vi "Martins HOT interface subtract and threshold.vi"() -> ()   [LabVIEW 2012]
uses:
  Sub VIs/Trap cluster.ctl
  <vilib>/vision/Image Controls.llb/IMAQ Image.ctl
  Sub VIs/Get measurement coordinates.vi
  <vilib>/Utility/inputDevices.llb/closeKeyboard.vi
  Sub VIs/Global variables.vi
  <vilib>/Utility/inputDevices.llb/keyboardAcquire.vi
  <vilib>/vision/driver/imaqhl.llb/IMAQ Grab Acquire.vi
  <vilib>/vision/driver/IMAQdx.llb/IMAQdx Grab.vi
  <vilib>/vision/driver/imaqll.llb/IMAQ Extract Buffer.vi
  <vilib>/Utility/file.llb/Write To Spreadsheet File (DBL).vi
  <vilib>/vision/driver/NI_Vision_Acquisition_Software.lvlib
  <vilib>/vision/NI_Vision_Development_Module.lvlib
panel:
  out "Measurement image":T1
  out "Monitoring image":T1
  in  "Apply Corrections":bool
  in  "View Licence":bool
  in  "ok":bool caption="Mark the center of \nthe spot using the \nzoom and the point\ntool, then click this \nbutton"
  in  "Stop program":bool
  in  "Updating trap cluster":bool
  out "Camera enabled":bool=TRUE
  out "SLM enabled":bool=TRUE
  in  "Run calibration":bool
  in  "Hologram generation":cluster{"Method":i32, "Iterations":i32}={"Method"=1, "Iterations"=50} {"Method" items=["Lenses & Gratings (3D)", " Gerchberg-Saxton (3D)", "Gerchberg-Saxton FFT (2D)"]}
  in  "Display hologram\nand computed \nimage plane":bool
  in  "ROI":T2={"Global Rectangle"=[709, 460, 1095, 702], "Contours"=[{"Contour Type"=0, "ROI Type"=1, "Points"=[709, 497]}, {"Contour Type"=0, "ROI Type"=1, "Points"=[1094, 460]}, {"Contour Type"=0, "ROI Type"=1, "Points"=[932, 701]}]}
  out "Monitor image":T1(plugin-control)
  in  "subtract\nbackground":bool
  in  "store \nbackground":bool
  in  "Update \nhologram\nsettings":bool
  in  "Coordinate mapping \n(Monitor to Measurement)":T3={"cZ"=1.0, "cY"=0.41527447, "cX"=-0.4158654, "sZ"=0.0, "sY"=-4.372315, "sX"=686.5264}
  in  "Transpose Measurement":bool
  out "Image\nsaturated":bool
  in  "Display ROIs":bool=TRUE
  out "Lost Frames":u32=1
  in  "Display ROIs":bool
  out "Using monitoring camera\nfor measurements":bool
  out "Global Report":T4={"Mean Value"=0.10129758, "Standard Variation"=1.6580093, "Minimal Value"=0.0, "Maximal Value"=146.0, "Area (calibrated)"=346800.0, "Area (pixels)"=346800, "%"=100.0, "Calibration Valid"=TRUE} {"Mean Value" format="%.2f"; "%" format="%.2f"; "Area (calibrated)" format="%.2f"; "Maximal Value" format="%.2f"; "Minimal Value" format="%.2f"; "Standard Variation" format="%.2f"}
  in  "Save image path":path=path "E:/David/SLM characterization/Measured data/120420 - Trapping" caption="start path"
  in  "save image":bool
  in  "Subtract \nthreshold":bool=TRUE
  in  "Edit trap cluster":bool
  in  "threshold":bool
  in  "Range":cluster{"Lower value":sgl, "Upper value":sgl}={"Lower value"=20.0, "Upper value"=255.0} {"Upper value" format="%.2f"; "Lower value" format="%.2f"}
  in  "Display data":bool
  in  "Measure \nintensities":bool
  in  "Purge data":bool
  in  "ROI size":dbl=50.0 min=2.0 step=2.0
  in  "Save data":bool
  in  "Record":bool
  out "Calculated image plane":dbl[][](graph)
  in  "G":bool[](array[boolean])=[FALSE, FALSE, FALSE]
  out "Current trap pos":T5={"X (IMAQ)"=[960.0, 563.0, 45.0], "Y (IMAQ)"=[282.0, 292.0, 975.0], "Z"=[0.0, 0.0, 0.0], "I"=[10.0, 10.0, 10.0], "Trap number"=[0, 1, 2], "ROI number"=[0, 1, 2], "Number of traps"=3, "Group"=[FALSE, FALSE, FALSE]}
  out "NI Vision error":errorcluster
  out "CUDA/SLM error":errorcluster
  in  "Cancel calibration":bool
  in  "Skip step if \ntimed out":bool
  in  "Display path":bool=TRUE
  out "Average step time (ms)":dbl=26.902770233568713
  in  "Step time \n(ms)":u32=20
  in  "Pause":bool
  in  "cancel path":bool
  out "Step skipped":bool
  in  "Path controls":T6={"follow path"=FALSE, "Step length"=0.1, "Arrive \nsimultaneously"=FALSE, "Synchronize traps"=FALSE, "Add current \npositions to path"=FALSE}
  in  "Create path":bool
  out "#":i32[](array[numeric])=[0, 1, 2]
  in  "Group \nTraps":bool
  in  "Move \nHandle":bool
  out "Displayed Hologram":u8[][](graph)
  in  "Coordinate mapping \n(IMAQ to SLM)":T3={"cZ"=1.0, "cY"=0.15274464, "cX"=0.15384616, "sZ"=0.0, "sY"=-91.72315, "sX"=-106.92308}
  in  "Transpose SLM":bool
  in  "I":dbl[](array[numeric])=[15.0, 15.0, 15.0]
  in  "Z":dbl[](array[numeric])=[0.0, 0.0, 0.0]
  in  "Max num of \nmeasurements":i32=-1
  # "Martin\nPersson 2011"
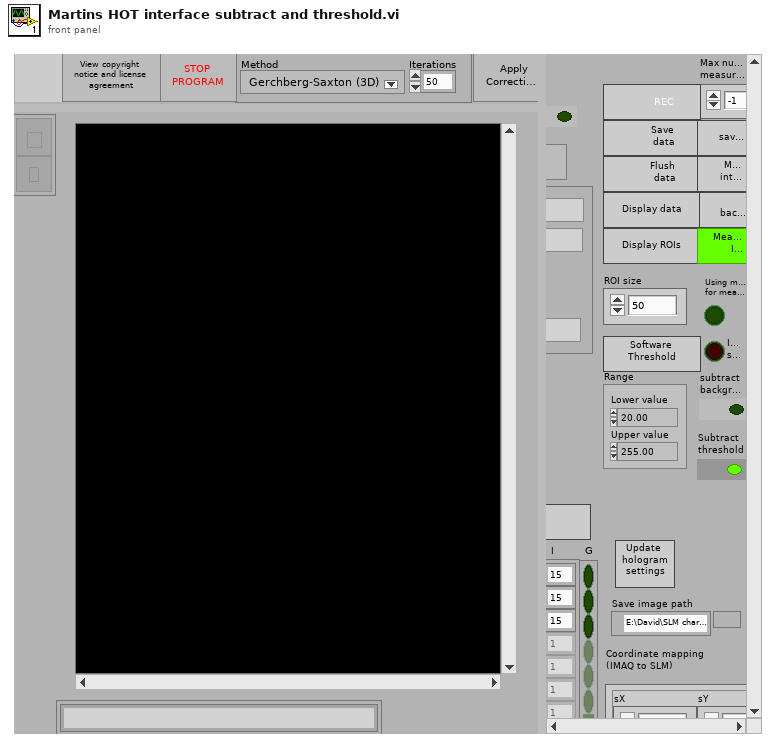
[diagram p1: front panel]
types:
  T1 = typedef "IMAQ Image.ctl" = refnum<image>
  T2 = cluster{"Global Rectangle":i32[], "Contours":cluster{"Contour Type":u32, "ROI Type":u32, "Points":i32[]}[]}
  T3 = cluster{"cZ":sgl, "cY":sgl, "cX":sgl, "sZ":sgl, "sY":sgl, "sX":sgl}
  T4 = cluster{"Mean Value":sgl, "Standard Variation":sgl, "Minimal Value":sgl, "Maximal Value":sgl, "Area (calibrated)":sgl, "Area (pixels)":u32, "%":sgl, "Calibration Valid":bool}
  T5 = typedef "Trap cluster.ctl" = cluster{"X (IMAQ)":sgl[], "Y (IMAQ)":sgl[], "Z":sgl[], "I":sgl[], "Trap number":i32[], "ROI number":i32[], "Number of traps":i32, "Group":bool[]}
  T6 = cluster{"follow path":bool, "Step length":dbl, "Arrive \nsimultaneously":bool, "Synchronize traps":bool, "Add current \npositions to path":bool}
  T7 = cluster{"CentroidX":dbl[], "CentroidY":dbl[], "I":dbl[], "Acquired Buffer Number":u32}
  T8 = enum16{"IMAQ (Camera Link)", "IMAQ ring", "IMAQdx (firewire)", "No camera"}
  T9 = typedef "IMAQdx.ctl" = refnum<k21>
  T10 = cluster{"Camera type":enum16{"IMAQ (Camera Link)", "IMAQ ring", "IMAQdx (firewire)", "No camera"}, "IMAQ Session":refnum<k11>, "IMAQdx Session":T9, "Image":T1, "Image buffers":T1[], "Camera error":errorcluster}
  T11 = typedef "Image Type" = u32
  T12 = cluster{"CentroidX":dbl[], "CentroidY":dbl[], "I":dbl[], "Acquired Buffer Number":u32}[]
  T13 = enum16{"Left Button", "Center Button", "Right Button", "Window Close"}
  T14 = typedef "ROI Descriptor" = cluster{"Global Rectangle":i32[], "Contours":cluster{"ID":enum32{"External", "Internal"}, "Type":u32, "Coordinates":i32[]}[]}
  T15 = enum16{"0", "1", "2", "3", "4", "5", "6", "7", "8", "9", "A", "B", "C", "D", "E", "F", "G", "H", "I", "J", "K", "L", "M", "N", "O", "P", "Q", "R", "S", "T", "U", "V", "W", "X", "Y", "Z", "F1", "F2", "F3", "F4", "F5", "F6", "F7", "F8", "F9", "F10", "F11", "F12", "F13", "F14", "F15", "ADD", "BACK", "BACKSLASH", "CAPITAL", "COMMA", "DECIMAL", "DELETE", "DIVIDE", "DOWN", "END", "EQUALS", "ESCAPE", "GRAVE (`)", "HOME", "INSERT", "LBRACKET", "LCONTROL", "LEFT", "L ALT", "LSHIFT", "LWIN", "MINUS", "MULTIPLY", "NEXT", "NUMLOCK", "NUMPAD_0", "NUMPAD_1", "NUMPAD_2", "NUMPAD_3", "NUMPAD_4", "NUMPAD_5", "NUMPAD_6", "NUMPAD_7", "NUMPAD_8", "NUMPAD_9", "PAUSE", "PERIOD", "PRIOR (PG UP)", "RBRACKET", "RCONTROL", "RETURN", "RIGHT", "R ALT", "RSHIFT", "RWIN", "SCROLL", "SEMICOLON", "SLASH", "SPACE", "SUBTRACT", "TAB", "UP", "ENTER (num pad)", "' (quote)"}[]
  T16 = typedef "LVRectTypeDef.ctl" = cluster{"Left":i16, "Top":i16, "Right":i16, "Bottom":i16}
  T17 = cluster{"Contour Type":u32, "ROI Type":u32, "Points":i32[]}[]
  T18 = cluster{"Contour Type":u32, "ROI Type":u32, "Points":i32[]}
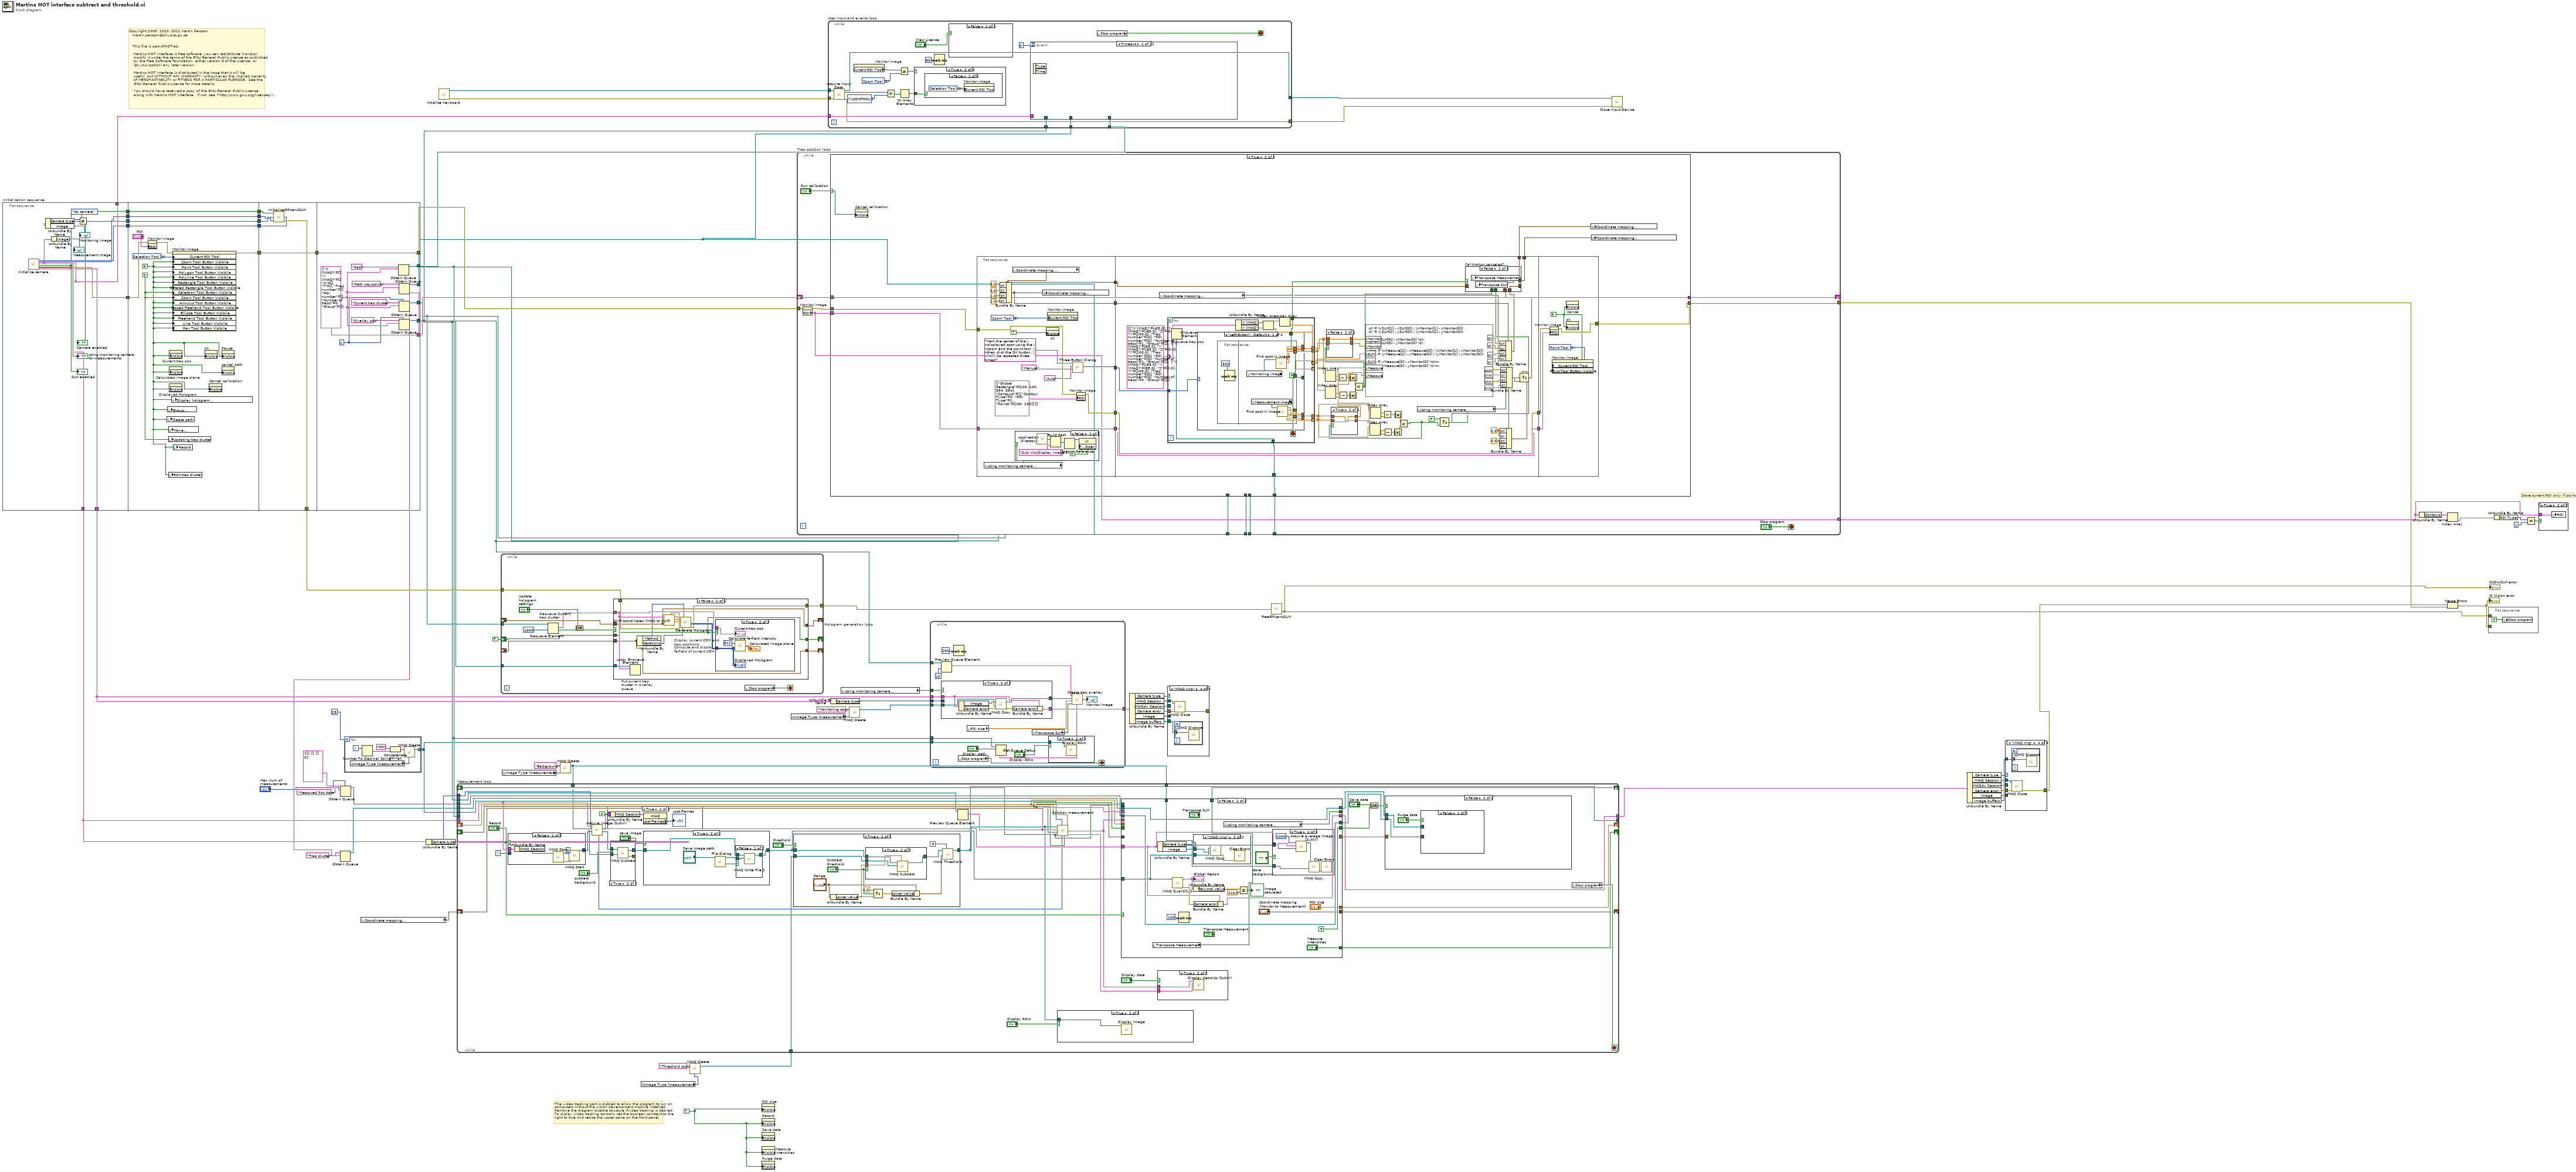
[diagram p0: block diagram]
diagram:
  w67 = TRUE ("Visible")
  # "Copyright 2009, 2010, 2011 Martin Persson \n   martin.persson@physics.gu.se\n\n\n   This file is part ofHOTlab.\n\n    Martins HOT interface is free software: you can redistribute it and/or \n    modify it under the terms of the GNU General Public License as published \n    by the Free Software Foundation, either version 3 of the License, or\n    (at your option) any later version.\n\n    Martins HOT interface is distributed in the hope that it will be \n    useful, but WITHOUT ANY WARRANTY; without even the implied warranty\n    of MERCHANTABILITY or FITNESS FOR A PARTICULAR PURPOSE.  See the\n    GNU General Public License for more details.\n\n    You should have received a copy of the GNU General Public License\n    along with Martins HOT interface.  If not, see <http://www.gnu.org/licenses/>."
  # "Store current ROI only if points"
  # "The video tracking part is disbled to allow the program to run on\ncomputers without the vision development module installed. \nRemove the diagram disable structure ifvideo tracking is desired. \nTo diplay video tracking controls, set the boolean constant to the \nright to true And resize the upper pane on the front panel."
  n1 = flat-sequence "Initialization sequence" {
    tunnel: [w82] -> w53
    tunnel: [w86] -> w52
    tunnel: [w85] -> w51
    tunnel: [w84] -> w50
    tunnel: [w83] -> w49
    tunnel: [w77] -> w26
    tunnel: [w75] -> w25
    tunnel: [w75] -> w37
    tunnel: w53 -> [w94]
    tunnel: w52 -> [w92]
    tunnel: w51 -> [w97]
    tunnel: w50 -> [w96]
    tunnel: w49 -> [w95]
    tunnel: [w94] -> w45
    tunnel: [w89] -> w44
    tunnel: [w97] -> w42
    tunnel: [w96] -> w41
    tunnel: [w95] -> w40
    tunnel: w45 -> [w100]
    tunnel: w44 -> [w103]
    tunnel: [w103] -> w43
    tunnel: w42 -> [w101]
    tunnel: w41 -> [w102]
    tunnel: w40 -> [w99]
    tunnel: [w98] -> w39
    tunnel: [w114] -> w48
    tunnel: w43 -> [w114]
    tunnel: [w112] -> w11
    tunnel: [w110] -> w47
    tunnel: [w108] -> w38
    tunnel: [w107] -> w12
    tunnel: [w104] -> w46
    frame #0 {
      n2 = call "Initialize camera.vi"() -> ("Use monitoring camera\nfor measurements"=→"Using monitoring camera\nfor measurements":bool, "Vision error out"=w86:errorcluster, "CUDA device ID"=w84:i32, "TrueFrame out"=w85:i32, "Measurement camera cluster"=w75:T10, "LUT path out"=w83:path, "SLM enabled"=w82:bool, "Monitoring camera cluster"=w77:T10)  [unwired: 3 in]
      "SLM enabled" <- w82
      n3 = Unbundle By Name(w77) -> ("Camera type"=w79:T8, "Image"=→"Monitoring image":T1)
      n4 = Unbundle By Name(w75) -> ("Image"=→"Measurement image":T1)
      n5 = Not Equal?(x=w79, y=T8."No camera") -> (x != y?=→"Camera enabled":bool)
    }
    frame #1 {
      w88 = TRUE ("ROI Tool Buttons Visibile:Zoom Tool Button Visible")
      w87 = FALSE ("ROI Tool Buttons Visibile:Zoom Tool Button Visible")
      w91 = u32 0 items=["Zoom Tool"=8, "Selection Tool"=0, "Pan Tool"=9, "Point Tool"=1, "Line Tool"=2, "Rectangle Tool"=3, "Rotated Rectangle Tool"=12, "Polyline Tool"=10, "Polygon Tool"=5, "Freehand Tool"=11, "Closed Freehand Tool"=6, "Ellipse Tool"=4, "Annulus Tool"=7] ("Current ROI Tool")
      n6 = property on="Monitor image" class="ImageControl"(error in=w92, "ROI"="ROI") -> (error out=w90:errorcluster)  [unwired: 1 in, 1 out]
      n7 = local write "Create path"(w87) -> ()
      n8 = local write "Group \nTraps"(w87) -> ()
      n9 = local write "Move \nHandle"(w87) -> ()
      n10 = local write "Updating trap cluster"(w88) -> ()
      n11 = local write "Edit trap cluster"(w87) -> ()
      n12 = property on="Current trap pos" class="Clust (strict)"("Visible"=w87) -> ()  [unwired: 2 in, 2 out]
      n13 = property on="Calculated image plane" class="IntGraph (strict)"("Visible"=w87) -> ()  [unwired: 2 in, 2 out]
      n14 = property on="Displayed Hologram" class="IntGraph (strict)"("Visible"=w87) -> ()  [unwired: 2 in, 2 out]
      n15 = local write "Display hologram\nand computed \nimage plane"(w87) -> ()
      n16 = property on="Monitor image" class="ImageControl"(error in=w90, "Current ROI Tool"=w91, "Zoom Tool Button Visibile"=w87, "Point Tool Button Visibile"=w87, "Polygon Tool Button Visibile"=w87, "Polyline Tool Button Visibile"=w87, "Rectangle Tool Button Visibile"=w87, "Rotated Rectangle Tool Button Visibile"=w87, "Selection Tool Button Visibile"=w88, "Zoom Tool Button Visibile"=w88, "Annulus Tool Button Visibile"=w87, "Closed Freehand Tool Button Visibile"=w87, "Ellipse Tool Button Visibile"=w87, "Freehand Tool Button Visibile"=w87, "Line Tool Button Visibile"=w87, "Pan Tool Button Visibile"=w87) -> (error out=w89:errorcluster)  [unwired: 1 in, 1 out]
      n17 = local write "Record"(w87) -> ()
      n18 = property on="ok" class="Bool"("Visible"=w87) -> ()  [unwired: 2 in, 2 out]
      n19 = property on="Cancel calibration" class="Bool"("Visible"=w87) -> ()  [unwired: 2 in, 2 out]
      n20 = property on="Pause" class="Bool (strict)"("Visible"=w87) -> ()  [unwired: 2 in, 2 out]
      n21 = property on="cancel path" class="Bool"("Visible"=w87) -> ()  [unwired: 2 in, 2 out]
    }
    frame #2 {
      n22 = call "InitializeGPUandSLM.vi"("TrueFrame"=w101, "deviceId"=w102, "Path to LUT file"=w99, "SLM enabled"=w100) -> ("CUDA/SLM error"=w98:errorcluster)  [unwired: 1 out]
    }
    frame #3 {
      w105 = 1 ("max queue size (-1, unlimited)")
      w104 = T5 {"X (IMAQ)"=[], "Y (IMAQ)"=[], "Z"=[], "I"=[], "Trap number"=[], "ROI number"=[], "Number of traps"=0, "Group"=[]} ("output cluster 2")
      n23 = Obtain Queue(name (unnamed)="Path", element data type=w104) -> (queue out=w112:refnum<queue>)  [unwired: 3 in, 2 out]
      n24 = Obtain Queue(name (unnamed)="Path waypoints", element data type=w104) -> (queue out=w110:refnum<queue>)  [unwired: 3 in, 2 out]
      n25 = Obtain Queue(max queue size (-1, unlimited)=w105, name (unnamed)="Current trap cluster", element data type=w104) -> (queue out=w108:refnum<queue>)  [unwired: 2 in, 2 out]
      n26 = Obtain Queue(max queue size (-1, unlimited)=w105, name (unnamed)="Overlay pos", element data type=w104) -> (queue out=w107:refnum<queue>)  [unwired: 2 in, 2 out]
    }
  }
  n27 = Obtain Queue(name (unnamed)="Trap cluster", element data type=w46) -> (queue out=w69:refnum<queue>)  [unwired: 3 in, 2 out]
  n28 = Obtain Queue(max queue size (-1, unlimited)="Max num of \nmeasurements", name (unnamed)="Measured Pos data", element data type=T7 {"CentroidX"=[], "CentroidY"=[], "I"=[], "Acquired Buffer Number"=0} ("Position data out")) -> (queue out=w71:refnum<queue>)  [unwired: 2 in, 2 out]
  n29 = for {
    N: 25 -> [_]
    tunnel: [w120] -> w10 mode=indexing
    i -> [w117]
    n30 = global read "Global variables.vi" "Image Type (measurement)"() -> (w115:T11)
    n31 = Number To Decimal String(number=w117) -> (decimal integer string=w116:string)  [unwired: 1 in]
    n32 = Concatenate Strings("ROI" ("Image Name"), w116) -> (w118:string)
    n33 = call "IMAQ Create"("Image Name"=w118, "Image Type"=w115) -> ("New Image"=w120:T1)  [unwired: 3 in, 1 out]
  }
  n34 = local read "Coordinate mapping \n(Monitor to Measurement)"() -> (w5:T3)
  n35 = Unbundle By Name(w25) -> ("Camera type"=w24:T8)
  n36 = call <vilib>:"Intialize Keyboard.vi"() -> ("error out"=w55:errorcluster, "device ID"=w73:refnum<k1>)  [unwired: 1 in, 9 out]
  n37 = while "Hologram generation loop" {
    tunnel: w38 -> [w134]
    tunnel: w12 -> [w132]
    tunnel: w39 -> [w130]
    tunnel: [w129] -> w35
    shift-right: [w128] -> _
    shift-left: _ -> [w127]
    shift-right: [w126] -> _
    shift-left: _ -> [w125]
    shift-right: [w122] -> _
    shift-left: FALSE ("Display hologram\nand computed \nimage plane") -> [w121]
    stop <- w135 stop-if-true
    n38 = Dequeue Element "Dequeue Current \ntrap cluster"(queue=w134, timeout in ms (-1)=1000) -> (element=w133:T5, timed out?=w131:bool)  [unwired: 1 in, 2 out]
    n39 = Or(x="Update \nhologram\nsettings", y=w131) -> (x .or. y?=w124:bool)
    n40 = case shown="False" w124 {
      tunnel: w127 -> [w141 _]
      tunnel: w133 -> [w145 _]
      tunnel: w132 -> [w144 _]
      tunnel: w130 -> [w143 w158]
      tunnel: [w142 w158] -> w129
      tunnel: [w141 "Coordinate mapping \n(IMAQ to SLM)"] -> w128
      tunnel: [w138 "Hologram generation"] -> w126
      tunnel: w125 -> [w138 _]
      tunnel: [w137 "Display hologram\nand computed \nimage plane"] -> w122
      tunnel: w121 -> [w137 _]
      frame False {
        n41 = Lossy Enqueue Element "Put current trap \ncluster in overlay \nqueue"(queue=w144, element=w145) -> ()  [unwired: 1 in, 4 out]
        n42 = Unbundle By Name(w138) -> ("Method"=w140:i32, "Iterations"=w139:i32)
        n43 = call "Shift coordinates (IMAQ to SLM).vi"("Trap cluster"=w145, "Coordinate mapping \n(IMAQ to SLM)"=w141) -> ("X (SLM)"=w146:sgl[], "Y (SLM)"=w149:sgl[], "Intensities"=w147:sgl[], "Z (SLM)"=w148:sgl[])  [unwired: 1 in, 1 out]
        n44 = call "Generate Hologram.vi"("x"=w146, "y"=w149, "z"=w148, "spot_intensities"=w147, "CUDA/SLM error in"=w143, "N_iterations"=w139, "method"=w140) -> ("CGH out"=w150:u8[][], "CUDA/SLM error out"=w142:errorcluster)  [unwired: 17 in, 2 out]
        n45 = case "Display current CGH and trap positions.\nCompute and display farfield of current CGH" shown="True" w137 {
          tunnel: w150 -> [_ w153]
          tunnel: w145 -> [_ w152]
          frame False {
          }
          frame True {
            n46 = call "Calculate farfield intensity.vi"("h_pSLM"=w153, "SLMsize"=512 ("Numeric")) -> ("Calculated image plane"=→"Calculated image plane":dbl[][])
            "Displayed Hologram" <- w153
            "Current trap pos" <- w152
          }
        }
      }
      frame True {
      }
    }
    n47 = local read "Stop program"() -> (w135:bool)
  }
  n48 = global read "Global variables.vi" "Image Type (measurement)"() -> (w3:T11)
  n49 = call "IMAQ Create"("Image Name"="Background", "Image Type"=w3) -> ("New Image"=w1:T1)  [unwired: 3 in, 1 out]
  n50 = global read "Global variables.vi" "Image Type (measurement)"() -> (w7:T11)
  n51 = call "IMAQ Create"("Image Name"="Threshold copy", "Image Type"=w7) -> ("New Image"=w9:T1)  [unwired: 3 in, 1 out]
  n52 = while "Measurement loop" {
    tunnel: w10 -> [w180]
    tunnel: w71 -> [w200]
    shift-right: [w199] -> _
    shift-left: _ -> [w178]
    tunnel: w69 -> [w198]
    shift-right: [w197] -> _
    shift-left: _ -> [w179]
    tunnel: [w181] -> _
    tunnel: w25 -> [w170]
    tunnel: w12 -> [w183]
    tunnel: w11 -> [_]
    tunnel: [w185] -> w29
    tunnel: w24 -> [w187]
    tunnel: w9 -> [w184]
    shift-right: [w174] -> _
    shift-left: w5 -> [w173]
    shift-right: [w165] -> _
    shift-left: _ -> [w164]
    tunnel: w1 -> [w163]
    tunnel: w1 -> [w160]
    i -> [w168]
    stop <- w201 stop-if-true
    n53 = case shown="False" "Record" {
      tunnel: w170 -> [w214 _]
      tunnel: [0 w215] -> w169
      tunnel: w168 -> [_ w215]
      frame False {
        n54 = Unbundle By Name(w214) -> ("IMAQ Session"=w213:refnum<k11>)
        n55 = call <vilib>:"IMAQ Stop.vi"("IMAQ Session In"=w213) -> ("error out"=w212:errorcluster, "IMAQ Session Out"=w211:refnum<k11>)  [unwired: 9 in]
        n56 = call <vilib>:"IMAQ Start.vi"("error in (no error)"=w212, "IMAQ Session In"=w211) -> ()  [unwired: 8 in, 2 out]
      }
      frame True {
      }
    }
    n57 = call "Acquire image (SubVI).vi"("Buffer number"=w169, "Camera type"=w187, "Measurement camera \ncluster in"=w170) -> ("Image Out"=w161:T1, "Measurement camera cluster out"=w186:T10, "Buffer Number Out"=w171:u32)  [unwired: 6 in]
    n58 = case shown="True" FALSE {
      tunnel: w186 -> [_ w207]
      frame False {
      }
      frame True {
        n59 = Unbundle By Name(w207) -> ("IMAQ Session"=w209:refnum<k11>)
        n60 = property class="IMAQ"(reference=w209) -> ("Lost Frames"=→"Lost Frames":u32)  [unwired: 1 in, 2 out]
      }
    }
    n61 = case shown="True" "subtract\nbackground" {
      tunnel: [w202 w206] -> w162
      tunnel: w161 -> [w202 w205]
      tunnel: w160 -> [_ w204]
      tunnel: [_ w203] -> _
      frame False {
      }
      frame True {
        n62 = call "IMAQ Subtract"("Image Src A"=w205, "Image Src B"=w204) -> ("Image Dst Out"=w206:T1, "error out"=w203:errorcluster)  [unwired: 5 in]
      }
    }
    n63 = case shown="True" "save image" {
      tunnel: w162 -> [w219 w224]
      tunnel: [w219 w223] -> w188
      frame False {
      }
      frame True {
        n64 = call "File Dialog"("start path"="Save image path") -> ("selected path"=w222:path, "cancelled"=w221:bool)  [unwired: 11 in, 2 out]
        n65 = case shown="False" w221 {
          tunnel: w224 -> [w227 w228]
          tunnel: [w226 w228] -> w223
          tunnel: w222 -> [w225 _]
          frame False {
            n66 = call-poly "IMAQ Write File 2"("File Path"=w225, "Image"=w227) -> ("Image Out (duplicate)"=w226:T1)  [unwired: 8 in, 1 out]
          }
          frame True {
          }
        }
      }
    }
    n67 = case shown="True" "threshold" {
      tunnel: w188 -> [w229 w237]
      tunnel: [w229 w235] -> w181
      tunnel: w184 -> [_ w230]
      frame False {
      }
      frame True {
        n68 = Unbundle By Name("Range") -> ("Lower value"=w231:sgl)
        n69 = case shown="True" "Subtract \nthreshold" {
          tunnel: w231 -> [_ w245]
          tunnel: w237 -> [w241 w244]
          tunnel: [w241 w243] -> w236
          tunnel: w230 -> [_ w242]
          frame False {
          }
          frame True {
            n70 = call "IMAQ Subtract"("Image Src A"=w244, "Constant"=w245, "Image Dst"=w242) -> ("Image Dst Out"=w243:T1)  [unwired: 4 in, 1 out]
          }
        }
        n71 = Select(t=sgl 0.0 ("Lower value"), s="Subtract \nthreshold", f=w231) -> (s? t:f=w234:sgl)
        n72 = Bundle By Name(cluster="Range", "Lower value"=w234) -> (w238:cluster{"Lower value":sgl, "Upper value":sgl})
        n73 = call "IMAQ Threshold"("Keep/Replace Value (Replace)"=FALSE, "Range"=w238, "Image Src"=w236) -> ("Image Dst Out"=w235:T1)  [unwired: 7 in, 1 out]
      }
    }
    n74 = Preview Queue Element(queue=w183) -> (element=w182:T5)  [unwired: 2 in, 3 out]
    n75 = call "Position measurement.vi"("Measure \nintensities"=w179, "ROI size"=w178, "Acquired Buffer Number"=w171, "Switch xy"=w164, "Coordinate mapping \n(Monitor to Measurement)"=w173, "ROIs"=w180, "Trap positions"=w182, "Image"=w181) -> ("Target coordinates"=w172:cluster{"X target":sgl[], "Y target":sgl[]}, "Position data out"=w176:T7)  [unwired: 1 in]
    n76 = case shown="True" "Display ROIs" {
      tunnel: w181 -> [_ w216]
      frame False {
      }
      frame True {
        n77 = call "Display Image.vi"("Image 2"=w216) -> ()  [unwired: 11 in]
      }
    }
    n78 = case shown="False" "Record" {
      tunnel: w200 -> [w266 w289]
      tunnel: [w266 w288] -> w196
      tunnel: [_ w287] -> w194
      tunnel: ["ROI size" w286] -> w199
      tunnel: w178 -> [_ w286]
      tunnel: w198 -> [w265 w285]
      tunnel: [w265 w284] -> w193
      tunnel: ["Measure \nintensities" w283] -> w197
      tunnel: w179 -> [_ w283]
      tunnel: [FALSE ("timed out?") w281] -> w190
      tunnel: w188 -> [w249 _]
      tunnel: w186 -> [w247 w280]
      tunnel: [w259 w280] -> w185
      tunnel: w182 -> [_ w279]
      tunnel: w176 -> [_ w278]
      tunnel: ["Coordinate mapping \n(Monitor to Measurement)" w277] -> w174
      tunnel: w173 -> [_ w277]
      tunnel: [w253 _] -> _
      tunnel: [w251 w276] -> w165
      tunnel: w164 -> [_ w276]
      tunnel: w163 -> [w248 _]
      frame False {
        n79 = local read "Transpose Measurement"() -> (w251:bool)
        n80 = Unbundle By Name(w247) -> ("Camera type"=w246:T8, "Image"=w252:T1)
        n81 = call "IMAQ Quantify 2"("Image"=w249) -> ("error out"=w260:errorcluster, "Global Report"=w258:T4)  [unwired: 8 in, 1 out]
        "Global Report" <- w258
        n82 = Wait (ms)(milliseconds to wait=u32 100) -> ()  [unwired: 1 out]
        n83 = case shown="\"IMAQ ring\"" w246 {
          tunnel: w249 -> [_ w275]
          tunnel: w252 -> [_ w274]
          frame "IMAQ (Camera Link)", Default {
          }
          frame "IMAQ ring" {
            n84 = call "IMAQ Copy"("Image Dst"=w274, "Image Src"=w275) -> ("error out"=w273:errorcluster)  [unwired: 4 in, 1 out]
            n85 = call <vilib>:"Clear Errors.vi"("error in (no error)"=w273) -> ()  [unwired: 6 in, 1 out]
          }
        }
        n86 = Unbundle By Name(w258) -> ("Maximal Value"=w257:sgl)
        n87 = Bundle By Name(cluster=w247, "Camera error"=w260) -> (w259:T10)
        n88 = local read "Using monitoring camera\nfor measurements"() -> (w253:bool)
        n89 = Greater Or Equal?(x=w257, y=sgl 210.0) -> (x >= y?=→"Image\nsaturated":bool)
        n90 = case shown="True" "store \nbackground" {
          tunnel: w248 -> [_ w271]
          tunnel: w247 -> [_ w270]
          tunnel: w246 -> [_ w269]
          frame False {
          }
          frame True {
            n91 = call "Acquire average image (SubVI).vi"("Camera type"=w269, "Measurement camera cluster in"=w270, "averaging time (ms)"=1000) -> ("Refnum out"=w267:T1)  [unwired: 8 in]
            n92 = call "IMAQ Copy"("Image Dst"=w271, "Image Src"=w267) -> ("error out"=w272:errorcluster)  [unwired: 4 in, 1 out]
            n93 = call <vilib>:"Clear Errors.vi"("error in (no error)"=w272) -> ()  [unwired: 6 in, 1 out]
          }
        }
      }
      frame True {
        n94 = Enqueue Element(queue=w285, element=w279) -> (queue out=w284:refnum<queue>)  [unwired: 2 in, 2 out]
        n95 = Enqueue Element(queue=w289, element=w278, timeout in ms (-1)=10000) -> (queue out=w288:refnum<queue>, timed out?=w281:bool, error out=w287:errorcluster)  [unwired: 1 in]
      }
    }
    n96 = case shown="True" "Display data" {
      tunnel: w176 -> [_ w218]
      tunnel: w172 -> [_ w217]
      frame False {
      }
      frame True {
        n97 = call "Display Cetroids (SubVI).vi"("Target coordinates"=w217, "Measurement data"=w218) -> ()  [unwired: 7 in, 3 out]
      }
    }
    n98 = Or(x="Save data", y=w190) -> (x .or. y?=w191:bool)
    n99 = case shown="False" w191 {
      tunnel: w196 -> [w291 w311]
      tunnel: w194 -> [_ w301]
      tunnel: w193 -> [w290 w300]
      frame False {
        n100 = case shown="False" "Purge data" {
          tunnel: w291 -> [_ w294]
          tunnel: w290 -> [_ w293]
          frame False {
          }
          frame True {
            n101 = Flush Queue(queue=w293) -> ()  [unwired: 1 in, 3 out]
            n102 = Flush Queue(queue=w294) -> ()  [unwired: 1 in, 3 out]
          }
        }
      }
      frame True {
        n103 = Flush Queue(queue=w311, error in (no error)=w301) -> (remaining elements=w307:T12)  [unwired: 2 out]
        n104 = Flush Queue(queue=w300, error in (no error)=w301) -> (remaining elements=w299:T5[])  [unwired: 2 out]
        n105 = for {
          tunnel: [w318] -> w310 mode=indexing
          tunnel: [w317] -> w309 mode=indexing
          tunnel: [w316] -> w302 mode=indexing
          tunnel: w307 -> [w315] mode=indexing
          tunnel: w299 -> [w314] mode=indexing
          tunnel: [w313] -> w298 mode=indexing
          tunnel: [w312] -> w297 mode=indexing
          workers-P: _ -> [_]
          n106 = Unbundle By Name(w315) -> ("CentroidX"=w318:dbl[], "CentroidY"=w317:dbl[], "Acquired Buffer Number"=w316:u32)
          n107 = Unbundle By Name(w314) -> ("X (IMAQ)"=w313:sgl[], "Y (IMAQ)"=w312:sgl[])
        }
        n108 = Transpose 2D Array(2D array=w310) -> (transposed array=w305:dbl[][])
        n109 = Transpose 2D Array(2D array=w309) -> (transposed array=w304:dbl[][])
        n110 = Transpose 2D Array(2D array=w298) -> (transposed array=w296:sgl[][])
        n111 = Transpose 2D Array(2D array=w297) -> (transposed array=w295:sgl[][])
        n112 = Build Array (concatenate)(w302, w305, w304, w296, w295) -> (w306:dbl[][])
        n113 = Transpose 2D Array(2D array=w306) -> (transposed array=w303:dbl[][])
        n114 = call-poly <vilib>:"Write To Spreadsheet File.vi"("format (%.3f)"="%.9f", "2D data"=w303) -> ()  [unwired: 6 in, 1 out]
      }
    }
    n115 = local read "Stop program"() -> (w201:bool)
  }
  n116 = property on="ROI size" class="DigNum (strict)"("Visible"=w67) -> ()  [unwired: 2 in, 2 out]
  n117 = property on="Record" class="Bool (strict)"("Visible"=w67) -> ()  [unwired: 2 in, 2 out]
  n118 = property on="Save data" class="Bool"("Visible"=w67) -> ()  [unwired: 2 in, 2 out]
  n119 = property on="Measure \nintensities" class="Bool (strict)"("Visible"=w67) -> ()  [unwired: 2 in, 2 out]
  n120 = property on="Purge data" class="Bool"("Visible"=w67) -> ()  [unwired: 2 in, 2 out]
  n121 = global read "Global variables.vi" "Image Type (measurement)"() -> (w6:T11)
  n122 = while "Trap position loop" {
    tunnel: w47 -> [w330]
    tunnel: w11 -> [w327]
    shift-right: [w329] -> _
    shift-left: w46 -> [w322]
    tunnel: w38 -> [w328]
    tunnel: w12 -> [w325]
    tunnel: [w324] -> w61
    tunnel: w48 -> [w321]
    tunnel: [w319] -> w59
    stop <- "Stop program" stop-if-true
    n123 = property on="Monitor image" class="ImageControl"(error in=w321) -> (error out=w320:errorcluster, "ROI"=w324:T2)  [unwired: 1 in, 1 out]
    n124 = case shown="True" "Run calibration" {
      selector: "Run calibration" -> [_ w534]
      tunnel: w330 -> [w356 _]
      tunnel: w322 -> [w355 w533]
      tunnel: [w334 w533] -> w329
      tunnel: w328 -> [w345 w542]
      tunnel: w327 -> [w343 _]
      tunnel: w325 -> [w340 _]
      tunnel: w324 -> [w339 w541]
      tunnel: w320 -> [w338 w538]
      tunnel: [w336 w535] -> w319
      frame False {
        n125 = case "Update trap cluster" shown="True" "Updating trap cluster" {
          tunnel: w355 -> [w358 w372]
          tunnel: [w358 w365] -> w346
          tunnel: w339 -> [_ w363]
          tunnel: w338 -> [w357 w362]
          tunnel: [w357 w361] -> w337
          frame False {
          }
          frame True {
            n126 = local read "Transpose SLM"() -> (w371:bool)
            n127 = call "Manage ROI.vi"("Switch X/Y"=w371, "Trap cluster in"=w372, "ROI in"=w363, "Group traps"="Group \nTraps") -> ("Replace ROI"=w359:bool, "ROI out"=w364:T2, "Previous ROI out"=w370:T2)
            n128 = case "Modify trap cluster for \ngroup or a single trap" shown="False" "Group \nTraps" {
              tunnel: [w382 w421] -> w365
              tunnel: w364 -> [w389 w422]
              tunnel: w372 -> [w388 w424]
              tunnel: w370 -> [_ w423]
              tunnel: "Z" -> [w387 w420]
              tunnel: "Move \nHandle" -> [_ w419]
              tunnel: w371 -> [w386 w418]
              tunnel: "I" -> [w384 w417]
              tunnel: "G" -> [w379 w416]
              frame False {
                n129 = case shown="True" "Edit trap cluster" {
                  tunnel: w389 -> [w400 w403]
                  tunnel: w388 -> [w399 w411]
                  tunnel: w387 -> [w398 _]
                  tunnel: w386 -> [w397 _]
                  tunnel: [w396 w410] -> w385
                  tunnel: w384 -> [w395 _]
                  tunnel: [w394 w409] -> w383
                  tunnel: [w393 w405] -> w382
                  tunnel: [w392 TRUE ("Update display")] -> w380
                  tunnel: w379 -> [w391 _]
                  tunnel: [w390 w407] -> w378
                  frame False {
                    n130 = call "ROI 2 Trap Cluster.vi"("Amplitudes"=w395, "Switch X/Y"=w397, "Group"=w391, "Trap Cluster in"=w399, "Z"=w398, "ROI"=w400) -> ("Group out"=w390:bool[], "Z out"=w396:dbl[], "Amplitudes out"=w394:dbl[], "Trap Cluster Out"=w393:T5, "Update display"=w392:bool)
                  }